vi "UHR-Fleezers Control (host) - 12.7e.vi"() -> ()   [LabVIEW 2012] (continued)
          tunnel: w4325 -> [w4338 w4370]
          tunnel: w4324 -> [w4337 w4369]
          tunnel: [w4336 w4368] -> w4322
          tunnel: [w4335 w4367] -> w4321
          tunnel: [w4333 w4354] -> w4319
          tunnel: [w4332 w4353] -> w4318
          tunnel: w4317 -> [w4333 w4359]
          tunnel: w4316 -> [w4332 w4362]
          tunnel: w4313 -> [_ _]
          frame False {
            w4334 = TRUE ("AI to FIFO")
            n2469 = xnode "Read/Write Control"("FPGA VI Reference In"=w4338, "error in"=w4337, "AI to FIFO"=w4334, "APD to FIFO"=w4334, "Start scan (MCL)"=w4334) -> ("FPGA VI Reference Out"=w4336:T20, "error out"=w4335:errorcluster)
          }
          frame True {
            w4366 = TRUE ("AI to FIFO")
            n2470 = local read "Scan steps (MCL)"() -> (w4345:u64)
            n2471 = local read "Scan lines (y)"() -> (w4341:u64)
            n2472 = local read "Fast Scan Dir"() -> (w4352:bool)
            n2473 = local read "Actual MCL Inc (V)"() -> (w4342:dbl)
            n2474 = Decrement(x=w4341) -> (x-1=w4340:u64)
            n2475 = Decrement(x=w4345) -> (x-1=w4344:u64)
            n2476 = Multiply(x=w4342, y=w4340) -> (x*y=w4339:dbl)
            n2477 = Divide(x=w4339, y=2.0) -> (x/y=w4349:dbl)
            n2478 = Multiply(x=w4342, y=w4344) -> (x*y=w4343:dbl)
            n2479 = Divide(x=w4343, y=2.0) -> (x/y=w4348:dbl)
            n2480 = Select(t=w4348, s=w4352, f=w4349) -> (s? t:f=w4347:dbl)
            n2481 = Select(t=w4349, s=w4352, f=w4348) -> (s? t:f=w4351:dbl)
            n2482 = Subtract(x=w4359, y=w4351) -> (x-y=w4350:dbl)
            n2483 = Subtract(x=w4362, y=w4347) -> (x-y=w4346:dbl)
            n2484 = local read "2D or 1D Scan"() -> (w4364:bool)
            n2485 = Not(x=w4352) -> (.not. x?=w4358:bool)
            n2486 = Not(x=w4364) -> (.not. x?=w4360:bool)
            n2487 = And(x=w4352, y=w4360) -> (x .and. y?=w4361:bool)
            n2488 = And(x=w4360, y=w4358) -> (x .and. y?=w4363:bool)
            n2489 = Select(t=w4362, s=w4363, f=w4346) -> (s? t:f=w4353:dbl)
            n2490 = Select(t=w4359, s=w4361, f=w4350) -> (s? t:f=w4354:dbl)
            n2491 = call "Volt to I16.vi"("Voltage In"=w4354) -> ("I16 Voltage Out"=w4357:i16)
            n2492 = call "Volt to I16.vi"("Voltage In"=w4353) -> ("I16 Voltage Out"=w4356:i16)
            n2493 = xnode "Read/Write Control"("FPGA VI Reference In"=w4370, "error in"=w4369, "AI to FIFO"=w4366, "APD to FIFO"=w4366, "Start scan (MCL)"=w4366, "AO1"=w4357, "AO2"=w4356) -> ("FPGA VI Reference Out"=w4368:T20, "error out"=w4367:errorcluster)
          }
        }
        "Initial Y" <- w4319
        "Initial X" <- w4318
        n2494 = local write "Tab Control 6"(T3."Imaging" ("Tab Control 6")) -> ()
        "wait to reset values" <- w4320
      }
    }
    n2495 = local read "APD Elements/DMA read"() -> (w3477:u32)
    n2496 = local read "Trap AI Elements/DMA read"() -> (w3694:u32)
    n2497 = xnode "Get APD Data"("FPGA VI Reference In"=w3633, "error in"=w3632, "Number of Elements"=w3477, "Timeout (ms)"=-1) -> ("Data"=w3663:u32[], "Elements Remaining"=→"APD FIFO Elements Remaining":u32)  [unwired: 2 out]
    n2498 = local read "Trap Pos Elements/DMA read"() -> (w3629:u32)
    n2499 = xnode "Invoke Method"("FPGA VI Reference In"=w3633, "error in"=w3632, "Number of Elements"=w3629, "Timeout (ms)"=-1) -> ("Data"=w3593:u16[], "Elements Remaining"=→"Trap Pos FIFO El Remaining":u32)  [unwired: 2 out]
    n2500 = xnode "Get Trap Data"("FPGA VI Reference In"=w3633, "error in"=w3632, "Number of Elements"=w3694, "Timeout (ms)"=-1 ("Timeout")) -> ("FPGA VI Reference Out"=w3528:T20, "error out"=w3527:errorcluster, "Data"=w3594:i16[], "Elements Remaining"=w3816:u32)
    "FIFO El. Rem." <- w3816
    n2501 = local read "DMA Update Period (s)"() -> (w3695:dbl)
    n2502 = local read "Trap AI FIFO Depth"() -> (w3818:u32)
    n2503 = local read "Number of APDs"() -> (w3496:u8)
    n2504 = Decimate 1D Array(w3593) -> (w3590:u16[], w3592:u16[], w3591:u16[])
    n2505 = feedback #6(0.0) -> (w3622:dbl)
    n2506 = Add(x=w3695, y=w3622) -> (x+y=w3792:dbl)
    n2507 = feedback-in #6(w3792) -> ()
    n2508 = To Time Stamp(1:w3622) -> (0:w3621:timestamp)
    n2509 = Subtract(x=w3818, y=w3694) -> (x-y=w3817:u32)
    n2510 = To Unsigned Long Integer(number=w3590) -> (unsigned 32bit integer=w3589:u32[])
    n2511 = Join Numbers(hi=w3592, lo=w3591) -> ((hi.lo)=w3588:u32[])
    n2512 = Divide(x=w3816, y=w3817) -> (x/y=w3815:dbl)
    "Buffer Status" <- w3815
    n2513 = case "Deinterlace APD signals" shown="3, Default" w3496 {
      tunnel: [w3828 w3834] -> w3476
      tunnel: w3663 -> [w3829 w3833]
      tunnel: [w3827 w3832] -> w3475
      tunnel: [w3826 w3830] -> w3462
      frame 3, Default {
        n2514 = Decimate 1D Array "APD signals"(w3829) -> (w3828:u32[], w3827:u32[], w3826:u32[])
      }
      frame 2 {
        n2515 = Decimate 1D Array "APD signals"(w3833) -> (w3834:u32[], w3832:u32[])
        n2516 = Multiply(x=w3832, y=u32 0) -> (x*y=w3830:u32[])
      }
    }
    n2517 = Join Numbers(hi=w3589, lo=w3588) -> ((hi.lo)=w3582:u64[])
    n2518 = call "IR AOM word to freq - vec.vi"("Frequency Word In (double vec)"=w3582) -> ("Frequency Out"=w3628:dbl[])
    n2519 = Equal?(x=w3815, y=1.0) -> (x = y?=w3813:bool)
    n2520 = case "Alert buffer overflow" shown="True" w3813 {
      frame False {
      }
      frame True {
        n2521 = call <vilib>:"Beep.vi"() -> ()  [unwired: 3 in, 9 out]
        "Overflow (data lost)" <- TRUE ("Overflow (data lost)")
      }
    }
    n2522 = Decimate 1D Array(w3628) -> (w3627:dbl[], w3626:dbl[])
    n2523 = Build Array(w3627, w3626) -> (w3625:dbl[][])
    n2524 = Bundle(w3476, w3475, w3462) -> (w3480:cluster{u32[], u32[], u32[]})  [unwired: 1 in]
    n2525 = Build Array(w3476, w3475, w3462) -> (w3753:u32[][])
    n2526 = for {
      tunnel: w3476 -> [w3824] mode=indexing
      n2527 = call "Smart Buffer (DBL) 1.vi"("new element [write]"=w3824, "mode"=T21."write") -> ()  [unwired: 4 in, 6 out]
    }
    n2528 = local read "APD Integration Time (s)"() -> (w3491:dbl)
    n2529 = To Double Precision Float(number=w3753) -> (double precision float=w3754:dbl[][])
    n2530 = feedback #7 "APD3"(w3462) -> (w3463:u32[])
    n2531 = feedback #8 "APD2"(w3475) -> (w3651:u32[])
    n2532 = feedback #9 "APD1"(w3476) -> (w3752:u32[])
    n2533 = Build Array (concatenate)(w3651, w3475) -> (w3650:u32[])
    n2534 = Build Array (concatenate)(w3463, w3462) -> (w3464:u32[])
    n2535 = Build Array (concatenate)(w3752, w3476) -> (w3749:u32[])
    n2536 = for {
      tunnel: w3475 -> [w3823] mode=indexing
      n2537 = call "Smart Buffer (DBL) 2.vi"("new element [write]"=w3823, "mode"=T21."write") -> ()  [unwired: 4 in, 6 out]
    }
    n2538 = Array Size(array=w3749) -> (size(s)=w3746:i32)
    n2539 = Array Size(array=w3476) -> (size(s)=w3748:i32)
    n2540 = Multiply(x=w3748, y="APD Ave N") -> (x*y=w3747:dbl)
    n2541 = Greater?(x=w3746, y=w3747) -> (0:w3750:bool)
    n2542 = Bundle("APD 1", "APD 2", "APD 3") -> (w3786:cluster{string, string, string})  [unwired: 1 out]
    n2543 = local read "Trap Sets"() -> (w3693:u32)
    n2544 = case shown="True" w3750 {
      tunnel: w3749 -> [w4126 w4135]
      tunnel: [w4126 w4133] -> w3700
      tunnel: w3747 -> [_ w4128]
      tunnel: w3746 -> [_ w4134]
      tunnel: w3650 -> [w4125 w4132]
      tunnel: [w4125 w4131] -> w3648
      tunnel: w3464 -> [w4124 w4130]
      tunnel: [w4124 w4127] -> w3492
      frame False {
      }
      frame True {
        n2545 = Subtract(x=w4134, y=w4128) -> (x-y=w4129:dbl)
        n2546 = Array Subset "APD3"(array=w4130, index=w4129, length=w4128) -> (w4127:u32[])
        n2547 = Array Subset "APD2"(array=w4132, index=w4129, length=w4128) -> (w4131:u32[])
        n2548 = Array Subset "APD1"(array=w4135, index=w4129, length=w4128) -> (w4133:u32[])
      }
    }
    n2549 = feedback-in #7(w3492) -> ()
    n2550 = feedback-in #8(w3648) -> ()
    n2551 = feedback-in #9(w3700) -> ()
    n2552 = Cluster To Array(cluster=w3786) -> (array=w3783:string[])
    n2553 = for "APD" {
      tunnel: w3754 -> [w4382] mode=indexing
      tunnel: w3491 -> [w4389]
      tunnel: [w4385] -> w3652 mode=indexing
      tunnel: "APD Disp. Scale" -> [w4386]
      tunnel: w3783 -> [w4384] mode=indexing
      tunnel: "APD Disp. Downsample" -> [w4380]
      tunnel: [w4383] -> w3782
      workers-P: _ -> [_]
      tunnel: w3621 -> [w4379]
      n2554 = call "integrate 1D array interval - double.vi"("Ave N"=w4380, "Array In"=w4382) -> ("Array Out"=w4381:dbl[])  [unwired: 1 out]
      n2555 = Multiply(x=w4389, y=w4380) -> (x*y=w4383:dbl)
      n2556 = Divide(x=w4381, y=w4386) -> (x/y=w4387:dbl[])
      n2557 = Bundle By Name("t0"=w4379, "Y"=w4387, "dt"=w4383) -> (w4388:waveform(dbl))  [unwired: 1 out]
      n2558 = Set Waveform Attribute(5:w4384, 6:"NI_ChannelName" ("name"), 7:w4388) -> (3:w4385:waveform(dbl))  [unwired: 1 in, 2 out]
    }
    "APD Display Period (s)" <- w3782
    n2559 = Reciprocal(x=w3782) -> (1/x=→"APD Display Freq. (Hz)":dbl)
    n2560 = case "Deinterlace trap data, average down PSD" shown="2" w3693 {
      tunnel: w3594 -> [w4407 w4472]
      tunnel: [w4404 w4469] -> w3686
      tunnel: [w4407 w4471] -> w3585
      tunnel: "Detector Type" -> [w4406 w4467]
      tunnel: [w4405 w4470] -> w3685
      tunnel: [w4403 w4468] -> w3790
      frame 1, Default {
        n2561 = Divide(x=w4407, y=3276.7) -> (x/y=w4408:dbl[])
        n2562 = Decimate 1D Array(w4408) -> (w4417:dbl[], w4416:dbl[], w4415:dbl[], w4414:dbl[], w4413:dbl[], w4412:dbl[], w4411:dbl[], w4410:dbl[])
        n2563 = case shown="\"IR-QPD + PSD + FB-QPD position\"" w4406 {
          tunnel: w4417 -> [w4441 w4466]
          tunnel: w4416 -> [w4440 w4465]
          tunnel: w4415 -> [w4425 w4443]
          tunnel: w4414 -> [w4426 w4453]
          tunnel: w4413 -> [w4439 w4464]
          tunnel: w4412 -> [w4438 w4463]
          tunnel: w4411 -> [w4422 w4444]
          tunnel: w4410 -> [w4421 w4442]
          tunnel: [w4420 w4450] -> w4405
          tunnel: [w4419 w4449] -> w4404
          tunnel: [w4418 w4448] -> w4403
          frame "IR-QPD + PSD + FB-QPD", Default {
            w4418 = 0  # Channel pattern
            n2564 = Divide(x=w4441, y=w4426) -> (x/y=w4428:dbl[])
            n2565 = Divide(x=w4440, y=w4426) -> (x/y=w4427:dbl[])
            n2566 = Divide(x=w4439, y=w4422) -> (x/y=w4424:dbl[])
            n2567 = Divide(x=w4438, y=w4421) -> (x/y=w4423:dbl[])
            n2568 = Build Array(w4428, w4427, w4426, w4425, w4424, w4423, w4422, w4421) -> (w4419:dbl[][])
            n2569 = Bundle("T1 Y", "T1 X", "T1 Sum", "FB Sum", "PSD Y", "PSD X", "PSD Y Sum", "PSD X Sum") -> (w4437:T44)  [unwired: 1 out]
            n2570 = Cluster To Array(cluster=w4437) -> (array=w4420:string[])
          }
          frame "IR-QPD + PSD + FB-QPD position" {
            w4448 = 3  # Channel pattern
            n2571 = Negate(x=w4444) -> (-x=w4445:dbl[])
            n2572 = Divide(x=w4466, y=w4453) -> (x/y=w4455:dbl[])
            n2573 = Divide(x=w4465, y=w4453) -> (x/y=w4454:dbl[])
            n2574 = Divide(x=w4464, y=w4444) -> (x/y=w4452:dbl[])
            n2575 = Divide(x=w4463, y=w4445) -> (x/y=w4451:dbl[])
            n2576 = Build Array(w4455, w4454, w4453, w4442, w4443, w4452, w4451, w4444) -> (w4449:dbl[][])
            n2577 = Bundle("T1 Y", "T1 X", "T1 Sum", "FB X", "FB Sum", "PSD Y", "PSD X", "PSD Y Sum") -> (w4462:T44)  [unwired: 1 out]
            n2578 = Cluster To Array(cluster=w4462) -> (array=w4450:string[])
          }
        }
      }
      frame 2 {
        n2579 = case shown="\"IR-QPD + PSD + FB-QPD X position\", Default" w4467 {
          tunnel: w4472 -> [w4534 w4606 w4677]
          tunnel: [w4473 w4597 w4608] -> w4471
          tunnel: [w4500 w4588 w4655] -> w4470
          tunnel: [w4499 w4551 w4622] -> w4469
          tunnel: [w4493 w4586 w4653] -> w4468
          frame "IR-QPD + PSD + FB-QPD" {
            w4493 = 1  # Channel pattern
            # "time average x2 the 4th signal and the 4 psd signals (detection laser)"
            # "deinterlace 3 signals from qpd"
            n2580 = Decimate 1D Array(w4534) -> (w4533:i16[], w4532:i16[], w4498:i16[], w4531:i16[], w4521:i16[], w4519:i16[], w4518:i16[], w4516:i16[])
            n2581 = Decimate 1D Array(w4498) -> (w4497:i16[], w4496:i16[])
            n2582 = Decimate 1D Array(w4533) -> (w4530:i16[], w4502:i16[])
            n2583 = Decimate 1D Array(w4532) -> (w4529:i16[], w4527:i16[])
            n2584 = Decimate 1D Array(w4531) -> (w4528:i16[], w4526:i16[])
            n2585 = call "downsample 1D array - double.vi"("Ave N"=2.0, "Array In"=w4521) -> ("Array Out"=w4520:dbl[])  [unwired: 1 out]
            n2586 = call "downsample 1D array - double.vi"("Ave N"=2.0, "Array In"=w4519) -> ("Array Out"=w4501:dbl[])  [unwired: 1 out]
            n2587 = call "downsample 1D array - double.vi"("Ave N"=2.0, "Array In"=w4518) -> ("Array Out"=w4517:dbl[])  [unwired: 1 out]
            n2588 = call "downsample 1D array - double.vi"("Ave N"=2.0, "Array In"=w4516) -> ("Array Out"=w4515:dbl[])  [unwired: 1 out]
            n2589 = Interleave 1D Arrays(w4530, w4529, w4528, w4502, w4527, w4526, w4497, w4496, w4520, w4501, w4517, w4515) -> (w4514:dbl[])
            n2590 = Divide(x=w4514, y=3276.7) -> (x/y=w4513:dbl[])
            n2591 = Decimate 1D Array(w4513) -> (w4512:dbl[], w4511:dbl[], w4510:dbl[], w4509:dbl[], w4508:dbl[], w4507:dbl[], w4495:dbl[], w4494:dbl[], w4506:dbl[], w4505:dbl[], w4504:dbl[], w4503:dbl[])
            n2592 = Divide(x=w4512, y=w4510) -> (x/y=w4480:dbl[])
            n2593 = Divide(x=w4511, y=w4510) -> (x/y=w4479:dbl[])
            n2594 = Divide(x=w4509, y=w4507) -> (x/y=w4478:dbl[])
            n2595 = Divide(x=w4508, y=w4507) -> (x/y=w4477:dbl[])
            n2596 = Divide(x=w4506, y=w4504) -> (x/y=w4476:dbl[])
            n2597 = Divide(x=w4505, y=w4503) -> (x/y=w4475:dbl[])
            n2598 = Build Array(w4480, w4479, w4510, w4478, w4477, w4507, w4495, w4494, w4476, w4475, w4504, w4503) -> (w4499:dbl[][])
            n2599 = Bundle("T1 Y", "T1 X", "T1 Sum", "T2 Y", "T2 X", "T2 Sum", "T1 FB Sum", "T2 FB Sum", "PSD Y", "PSD X", "PSD Y Sum", "PSD X Sum") -> (w4481:T45)  [unwired: 1 out]
            n2600 = To Word Integer(number=w4514) -> (16bit integer=w4473:i16[])
            n2601 = Cluster To Array(cluster=w4481) -> (array=w4500:string[])
          }
          frame "IR-QPD + PSD + FB-QPD X position", Default {
            w4586 = 2  # Channel pattern
            # "time average x2 the 3 psd signals (detection laser)"
            # "deinterlace 3 signals from qpds"
            n2602 = Decimate 1D Array(w4606) -> (w4605:i16[], w4604:i16[], w4587:i16[], w4603:i16[], w4549:i16[], w4546:i16[], w4543:i16[], w4574:i16[])
            n2603 = Select(t=i16 -1, s="Flip X Sign", f=i16 1) -> (s? t:f=w4539:i16)
            n2604 = Multiply(x=w4604, y=w4539) -> (x*y=w4540:i16[])
            n2605 = Decimate 1D Array(w4587) -> (w4572:i16[], w4570:i16[])
            n2606 = Decimate 1D Array(w4605) -> (w4602:i16[], w4589:i16[])
            n2607 = Decimate 1D Array(w4540) -> (w4601:i16[], w4599:i16[])
            n2608 = Decimate 1D Array(w4603) -> (w4600:i16[], w4598:i16[])
            n2609 = Decimate 1D Array(w4574) -> (w4573:i16[], w4571:i16[])
            n2610 = call "downsample 1D array - I16.vi"("Ave N"=2.0, "Array In"=w4549) -> ("Array Out"=w4547:i16[])  [unwired: 1 in]
            n2611 = call "downsample 1D array - I16.vi"("Ave N"=2.0, "Array In"=w4543) -> ("Array Out"=w4541:i16[])  [unwired: 1 in]
            n2612 = call "downsample 1D array - I16.vi"("Ave N"=2.0, "Array In"=w4546) -> ("Array Out"=w4544:i16[])  [unwired: 1 in]
            n2613 = Interleave 1D Arrays(w4602, w4601, w4600, w4589, w4599, w4598, w4573, w4572, w4571, w4570, w4547, w4544, w4541) -> (w4597:i16[])
            n2614 = Divide(x=w4597, y=3276.7) -> (x/y=w4596:dbl[])
            n2615 = Decimate 1D Array(w4596) -> (w4595:dbl[], w4594:dbl[], w4593:dbl[], w4592:dbl[], w4591:dbl[], w4590:dbl[], w4562:dbl[], w4560:dbl[], w4559:dbl[], w4557:dbl[], w4556:dbl[], w4555:dbl[], w4552:dbl[])
            n2616 = Negate(x=w4552) -> (-x=w4550:dbl[])
            n2617 = Divide(x=w4556, y=w4552) -> (x/y=w4554:dbl[])
            n2618 = Divide(x=w4555, y=w4550) -> (x/y=w4553:dbl[])
            n2619 = Divide(x=w4595, y=w4593) -> (x/y=w4578:dbl[])
            n2620 = Divide(x=w4594, y=w4593) -> (x/y=w4577:dbl[])
            n2621 = Divide(x=w4592, y=w4590) -> (x/y=w4576:dbl[])
            n2622 = Divide(x=w4591, y=w4590) -> (x/y=w4575:dbl[])
            n2623 = Divide(x=w4562, y=w4560) -> (x/y=w4561:dbl[])
            n2624 = Divide(x=w4559, y=w4557) -> (x/y=w4558:dbl[])
            n2625 = Build Array(w4578, w4577, w4593, w4576, w4575, w4590, w4561, w4560, w4558, w4557, w4554, w4553, w4552) -> (w4551:dbl[][])
            n2626 = Bundle("T1 Y", "T1 X", "T1 Sum", "T2 Y", "T2 X", "T2 Sum", "T1 FB X", "T1 FB Sum", "T2 FB X", "T2 FB Sum", "PSD Y", "PSD X", "PSD Y Sum") -> (w4579:T46)  [unwired: 1 out]
            n2627 = Cluster To Array(cluster=w4579) -> (array=w4588:string[])
          }
          frame "IR-QPD + PSD + FB-QPD XY positions" {
            w4653 = 4  # Channel pattern
            # "time average x2 the 3 psd signals (detection laser)"
            # "deinterlace 3 signals from qpds"
            n2628 = Decimate 1D Array(w4677) -> (w4676:i16[], w4675:i16[], w4654:i16[], w4674:i16[], w4620:i16[], w4666:i16[], w4665:i16[], w4642:i16[])
            n2629 = Decimate 1D Array "Feedback Sum"(w4654) -> (w4638:i16[], w4636:i16[])
            n2630 = Decimate 1D Array "QPD Y"(w4676) -> (w4673:i16[], w4656:i16[])
            n2631 = Decimate 1D Array "QPD X"(w4675) -> (w4672:i16[], w4670:i16[])
            n2632 = Decimate 1D Array "Feedback Y"(w4620) -> (w4619:i16[], w4618:i16[])
            n2633 = Decimate 1D Array "QPD Sum"(w4674) -> (w4671:i16[], w4669:i16[])
            n2634 = Decimate 1D Array "Feedback X"(w4642) -> (w4639:i16[], w4637:i16[])
            n2635 = call "downsample 1D array - double.vi"("Ave N"=2.0, "Array In"=w4666) -> ("Array Out"=w4641:dbl[])  [unwired: 1 out]
            n2636 = call "downsample 1D array - double.vi"("Ave N"=2.0, "Array In"=w4665) -> ("Array Out"=w4640:dbl[])  [unwired: 1 out]
            n2637 = Interleave 1D Arrays(w4673, w4672, w4671, w4656, w4670, w4669, w4619, w4639, w4638, w4618, w4637, w4636, w4641, w4640) -> (w4664:dbl[])
            n2638 = Divide(x=w4664, y=3276.7) -> (x/y=w4663:dbl[])
            n2639 = Decimate 1D Array(w4663) -> (w4662:dbl[], w4661:dbl[], w4660:dbl[], w4659:dbl[], w4658:dbl[], w4657:dbl[], w4615:dbl[], w4629:dbl[], w4613:dbl[], w4614:dbl[], w4627:dbl[], w4611:dbl[], w4625:dbl[], w4623:dbl[])
            n2640 = Negate(x=w4623) -> (-x=w4621:dbl[])
            n2641 = Divide(x=w4625, y=w4621) -> (x/y=w4624:dbl[])
            n2642 = Divide(x=w4614, y=w4611) -> (x/y=w4610:dbl[])
            n2643 = Divide(x=w4615, y=w4613) -> (x/y=w4612:dbl[])
            n2644 = Divide(x=w4662, y=w4660) -> (x/y=w4646:dbl[])
            n2645 = Divide(x=w4661, y=w4660) -> (x/y=w4645:dbl[])
            n2646 = Divide(x=w4659, y=w4657) -> (x/y=w4644:dbl[])
            n2647 = Divide(x=w4658, y=w4657) -> (x/y=w4643:dbl[])
            n2648 = Divide(x=w4629, y=w4613) -> (x/y=w4628:dbl[])
            n2649 = Divide(x=w4627, y=w4611) -> (x/y=w4626:dbl[])
            n2650 = Build Array(w4646, w4645, w4660, w4644, w4643, w4657, w4612, w4628, w4613, w4610, w4626, w4611, w4624, w4623) -> (w4622:dbl[][])
            n2651 = Bundle("T1 Y", "T1 X", "T1 Sum", "T2 Y", "T2 X", "T2 Sum", "T1 FB Y", "T1 FB X", "T1 FB Sum", "T2 FB Y", "T2 FB X", "T2 FB Sum", "PSD X", "PSD Y Sum") -> (w4609:T47)  [unwired: 1 out]
            n2652 = To Word Integer(number=w4664) -> (16bit integer=w4608:i16[])
            n2653 = Cluster To Array(cluster=w4609) -> (array=w4655:string[])
          }
        }
      }
    }
    "AI labels" <- w3685
    n2654 = local read "APD Integration Time (s)"() -> (w3658:dbl)
    n2655 = Array Size(array=w3700) -> (size(s)=w3745:i32)
    n2656 = call <vilib>:"Std Deviation and Variance.vi"("X"=w3648) -> ("standard deviation"=w3647:dbl)  [unwired: 1 in, 2 out]
    n2657 = Add Array Elements(numeric array=w3648) -> (sum=w3649:u32)
    n2658 = Add Array Elements(numeric array=w3700) -> (sum=w3755:u32)
    n2659 = call <vilib>:"Std Deviation and Variance.vi"("X"=w3700) -> ("standard deviation"=w3699:dbl)  [unwired: 1 in, 2 out]
    n2660 = Divide(x=w3647, y=w3491) -> (x/y=w3644:dbl)
    "Rate sigma (Hz) 2" <- w3644
    n2661 = Multiply(x=w3491, y=w3745) -> (x*y=w3493:dbl)
    "Int. Time (s)" <- w3493
    n2662 = Divide(x=w3649, y=w3493) -> (x/y=w3645:dbl)
    "APD 2 Rate (Hz)" <- w3645
    n2663 = Multiply(x="APD Disp. Scale", y=w3652) -> (x*y=w3660:waveform(dbl)[])
    n2664 = Divide(x=w3755, y=w3493) -> (x/y=w3697:dbl)
    "APD 1 Rate (Hz)" <- w3697
    n2665 = Divide(x=w3699, y=w3491) -> (x/y=w3698:dbl)
    "Rate sigma (Hz)" <- w3698
    n2666 = Divide(x=w3644, y=w3645) -> (x/y=→"Sigma/Mean 2":dbl)
    n2667 = Multiply(x="APD Disp. Downsample", y=w3658) -> (x*y=w3656:dbl)
    n2668 = Divide(x=w3698, y=w3697) -> (x/y=→"Sigma/Mean":dbl)
    n2669 = Divide(x=w3660, y=w3656) -> (x/y=w3483:waveform(dbl)[])
    n2670 = Index Array(array=w3483, index=0) -> (element=w3641:waveform(dbl))
    n2671 = Index Array(array=w3483, index=1) -> (element=w3639:waveform(dbl))
    n2672 = Index Array(array=w3483, index=2) -> (element=w3485:waveform(dbl))
    n2673 = Subtract(x=w3641, y="APD 1 Offset") -> (x-y=w3637:waveform(dbl))
    n2674 = Subtract(x=w3639, y="APD 2 Offset") -> (x-y=w3636:waveform(dbl))
    n2675 = Subtract(x=w3485, y="APD 3 Offset") -> (x-y=w3482:waveform(dbl))
    n2676 = Add Array Elements(numeric array=w3492) -> (sum=w3495:u32)
    n2677 = call <vilib>:"Std Deviation and Variance.vi"("X"=w3492) -> ("standard deviation"=w3494:dbl)  [unwired: 1 in, 2 out]
    n2678 = Build Array(w3637, w3636, w3482) -> (→"APD Chart":waveform(dbl)[])
    n2679 = Divide(x=w3495, y=w3493) -> (x/y=w3489:dbl)
    "APD 3 Rate (Hz)" <- w3489
    n2680 = Divide(x=w3494, y=w3491) -> (x/y=w3490:dbl)
    "Rate sigma (Hz) 3" <- w3490
    n2681 = Divide(x=w3490, y=w3489) -> (x/y=→"Sigma/Mean 3":dbl)
    n2682 = local read "Data Period (s)"() -> (w3544:dbl)
    n2683 = local read "BD 1 Frequency 2 (MHz)"() -> (w3577:dbl)
    n2684 = local read "BD 1 Frequency 1 (MHz)"() -> (w3578:dbl)
    n2685 = Decimate 1D Array(w3585) -> (w3609:i16[], w3608:i16[], w3606:i16[], w3605:i16[])  [unwired: 9 out]
    n2686 = Multiply(x=w3544, y="Trap Pos. Disp. Downsample") -> (x*y=w3542:dbl)
    n2687 = Divide(x=w3609, y=w3608) -> (x/y=w3610:dbl[])
    n2688 = Divide(x=w3606, y=w3605) -> (x/y=w3607:dbl[])
    n2689 = local read "AOM X Cal (nm/MHz)"() -> (w3575:dbl)
    n2690 = Split 1D Array(array=w3610, index="N El. to Ave.") -> (second subarray=w3613:dbl[])  [unwired: 1 out]
    n2691 = Split 1D Array(array=w3607, index="N El. to Ave.") -> (second subarray=w3612:dbl[])  [unwired: 1 out]
    n2692 = Multiply(x=w3544, y="Trap Disp. Downsample") -> (x*y=w3623:dbl)
    "Display Period (s)" <- w3623
    n2693 = for "Trap AI" {
      tunnel: [w4402] -> w3469 mode=indexing
      tunnel: w3621 -> [w4393]
      tunnel: "Trap Disp. Downsample" -> [w4400]
      tunnel: w3686 -> [w4398] mode=indexing
      tunnel: w3544 -> [w4397]
      tunnel: w3685 -> [w4396] mode=indexing
      tunnel: [w4395] -> w3655 mode=indexing
      tunnel: w3623 -> [w4394]
      workers-P: _ -> [_]
      n2694 = Bundle By Name("Y"=w4398, "dt"=w4397) -> (w4399:waveform(dbl))  [unwired: 1 out]
      n2695 = Set Waveform Attribute(5:w4396, 6:"NI_ChannelName" ("name"), 7:w4399) -> (3:w4395:waveform(dbl))  [unwired: 1 in, 2 out]
      n2696 = call "downsample 1D array - double.vi"("Ave N"=w4400, "Array In"=w4398) -> ("Array Out"=w4401:dbl[])  [unwired: 1 out]
      n2697 = Bundle By Name(cluster=w4395, "t0"=w4393, "Y"=w4401, "dt"=w4394) -> (w4402:waveform(dbl))
    }
    n2698 = Bundle("BD 1 Frequency 1 (MHz)"=w3578, "BD 1 Frequency 2 (MHz)"=w3577) -> (w3579:T48)  [unwired: 1 out]
    n2699 = call-poly <vilib>:"Mean.vi"("X"=w3612) -> ("mean"=w3600:dbl)  [unwired: 1 out]
    n2700 = call-poly <vilib>:"Mean.vi"("X"=w3613) -> ("mean"=w3601:dbl)  [unwired: 1 out]
    n2701 = Reciprocal(x=w3623) -> (1/x=→"Trap Disp. Freq. (Hz)":dbl)
    n2702 = Cluster To Array(cluster=w3579) -> (array=w3576:dbl[])
    n2703 = local read "Trap X AI1 (DMA)"() -> (w3611:T13)
    n2704 = local read "Data points/scans (MCL)"() -> (w3765:dbl)
    n2705 = To Fixed-Point(number=w3600) -> (fixed-point=w3598:fxp<+/-,16,1>)  [unwired: 1 in]
    n2706 = To Fixed-Point(number=w3601) -> (fixed-point=w3599:fxp<+/-,16,1>)  [unwired: 1 in]
    n2707 = Bundle("Trap 1 Pos.", "Trap 2 Pos.") -> (w3620:cluster{string, string})  [unwired: 1 out]
    n2708 = Bundle By Name(cluster=w3611, "Set 1"=w3599, "Set 2"=w3598) -> (→"Trap X AI1 (DMA)":T13)
    n2709 = Cluster To Array(cluster=w3620) -> (array=w3617:string[])
    n2710 = Unbundle(w3480) -> (w3481:u32[])  [unwired: 2 out]
    n2711 = Select(t=-1.0, s="Negate Y Axis", f=1.0) -> (s? t:f=w3561:dbl)
    n2712 = for "Trap Position" {
      tunnel: w3625 -> [w3994] mode=indexing
      tunnel: "Trap Pos. Disp. Downsample" -> [w3993]
      tunnel: w3542 -> [w3991]
      tunnel: w3621 -> [w3990]
      tunnel: w3617 -> [w3988] mode=indexing
      tunnel: [w3987] -> w3531 mode=indexing
      tunnel: w3576 -> [w3985] mode=indexing
      tunnel: w3575 -> [w3983]
      tunnel: w3561 -> [w3982]
      n2713 = call "downsample 1D array - double.vi"("Ave N"=w3993, "Array In"=w3994) -> ("Array Out"=w3992:dbl[])  [unwired: 1 out]
      n2714 = Subtract(x=w3992, y=w3985) -> (x-y=w3986:dbl[])
      n2715 = Multiply(x=w3983, y=w3986) -> (x*y=w3984:dbl[])
      n2716 = Multiply(x=w3982, y=w3984) -> (x*y=w3981:dbl[])
      n2717 = Bundle By Name("Y"=w3981, "dt"=w3991, "t0"=w3990) -> (w3989:waveform(dbl))  [unwired: 1 out]
      n2718 = Set Waveform Attribute(5:w3988, 6:"NI_ChannelName" ("name"), 7:w3989) -> (3:w3987:waveform(dbl))  [unwired: 1 in, 2 out]
    }
    n2719 = To Double Precision Float(number=w3481) -> (double precision float=w3683:dbl[])
    n2720 = local read "Display Period (s)"() -> (w3672:dbl)
    n2721 = Increment(x=w3765) -> (x+1=w3766:dbl)
    n2722 = Index Array(array=w3531, index=0) -> (element=w3535:waveform(dbl))
    n2723 = Index Array(array=w3531, index=1) -> (element=w3530:waveform(dbl))
    n2724 = feedback #10(w3766) -> (w3769:dbl)
    n2725 = Select(t=0, s=w3756, f=w3769) -> (s? t:f=w3762:dbl)
    n2726 = Array Size(array=w3683) -> (size(s)=w3768:i32)
    n2727 = Build Array (concatenate)(w3652, w3469) -> (w3474:waveform(dbl)[])
    "All Signals" <- w3474
    n2728 = Add(x=w3768, y=w3762) -> (x+y=w3763:dbl)
    n2729 = Unbundle By Name(w3535) -> ("Y"=w3536:dbl[])
    n2730 = Divide(x="Bead Sep. Int. Time (s)", y=w3672) -> (x/y=w3571:dbl)
    n2731 = Add(x=w3536, y="FB Trap Pos Offset") -> (x+y=w3534:dbl[])
    "T1 x pos data" <- w3534
    n2732 = Greater?(x=w3763, y=w3765) -> (0:w3764:bool)
    n2733 = feedback #11(w3534) -> (w3573:dbl[])
    n2734 = Build Array (concatenate)(w3534, w3573) -> (w3572:dbl[])
    n2735 = Bundle By Name(cluster=w3535, "Y"=w3534) -> (w3533:waveform(dbl))
    n2736 = Select(t=w3762, s=w3764, f=w3763) -> (s? t:f=w3761:dbl)
    n2737 = feedback-in #10(w3761) -> ()
    n2738 = local read "MCL Scanning"() -> (w3759:bool)
    n2739 = Bundle(w3533, w3530) -> (w3529:cluster{waveform(dbl), waveform(dbl)})  [unwired: 1 out]
    n2740 = Index Array(array=w3469, index="index 1") -> (element=w3468:waveform(dbl))
    n2741 = Index Array(array=w3469, index="index 2") -> (element=w3473:waveform(dbl))
    n2742 = Split 1D Array(array=w3572, index=w3571) -> (first subarray=w3565:dbl[])  [unwired: 1 out]
    n2743 = feedback-in #11(w3565) -> ()
    n2744 = Unbundle By Name(w3468) -> ("Y"=w3467:dbl[])
    n2745 = Unbundle By Name(w3473) -> ("Y"=w3472:dbl[])
    n2746 = Not(x=w3764) -> (.not. x?=w3758:bool)
    n2747 = Cluster To Array(cluster=w3529) -> (array=w3505:waveform(dbl)[])
    "Trap Positions" <- w3505
    n2748 = call-poly <vilib>:"Mean.vi"("X"=w3565) -> ("mean"=w3564:dbl)  [unwired: 1 out]
    "Mean T1 Position (nm)" <- w3564
    n2749 = Subtract(x=w3565, y=w3564) -> (x-y=w3570:dbl[])
    n2750 = Square(x=w3570) -> (x^2=w3569:dbl[])
    n2751 = And(x=w3758, y=w3759) -> (x .and. y?=w3760:bool)
    n2752 = call-poly <vilib>:"Mean.vi"("X"=w3569) -> ("mean"=w3568:dbl)  [unwired: 1 out]
    n2753 = call-poly <vilib>:"Mean.vi"("X"=w3467) -> ("mean"=→"Trap 1 sum mean":dbl)  [unwired: 1 out]
    n2754 = call-poly <vilib>:"Mean.vi"("X"=w3472) -> ("mean"=→"Trap 2 sum mean":dbl)  [unwired: 1 out]
    n2755 = Square Root(x=w3568) -> (sqrt(x)=w3567:dbl)
    n2756 = Or(x=w3760, y=w3756) -> (x .or. y?=w3757:bool)
    n2757 = Equal?(x="Tab Control 6", y=T38."High Res Display") -> (x = y?=w3689:bool)
    n2758 = Multiply(x=10.0, y=w3567) -> (x*y=→"Trap 1 Position RMS (A)":dbl)
    n2759 = case "For displaying the high resolution display (no downsampling)" shown="True" w3689 {
      tunnel: w3655 -> [_ w4014]
      frame False {
      }
      frame True {
        n2760 = Index Array(array=w4014, index="High Res. Display") -> (element=w4015:waveform(dbl))
        n2761 = call <vilib>:"Std Deviation and Variance.vi"("X"=w4015) -> ("mean"=w4022:dbl, "standard deviation"=w4027:dbl)  [unwired: 1 in, 1 out]
        "Mean Intensity" <- w4022
        "Sigma" <- w4027
        n2762 = Subtract(x=w4015, y=w4022) -> (x-y=w4021:waveform(dbl))
        n2763 = Select(t=w4021, s="Subtract mean", f=w4015) -> (s? t:f=→"1 Channel":waveform(dbl))
        n2764 = Divide(x=w4027, y=w4022) -> (x/y=→"Sigma/Mean":dbl)
        n2765 = feedback #12(1) -> (w4016:i32)
        n2766 = Greater Or Equal?(x=w4016, y="Slow mean N ave.") -> (x >= y?=w4029:bool)
        n2767 = Increment(x=w4016) -> (x+1=w4031:i32)
        n2768 = Select(t=1, s=w4029, f=w4031) -> (s? t:f=w4018:i32)
        n2769 = feedback-in #12(w4018) -> ()
        n2770 = feedback #13() -> (w4019:waveform(dbl))  [unwired: 1 out]
        n2771 = case shown="Default" w4016 {
          tunnel: [w4034 w4037] -> w4020
          tunnel: w4019 -> [w4036 _]
          tunnel: w4015 -> [w4035 w4037]
          frame Default {
            n2772 = call-poly <vilib>:"Append Waveforms.vi"("waveform B"=w4035, "waveform A"=w4036) -> ("waveform out"=w4034:waveform(dbl))  [unwired: 1 in, 8 out]
          }
          frame 1 {
          }
        }
        n2773 = feedback-in #13(w4020) -> ()
        n2774 = case shown="True" w4029 {
          tunnel: w4020 -> [_ w4033]
          frame False {
          }
          frame True {
            n2775 = call-poly <vilib>:"Mean.vi"("X"=w4033) -> ("mean"=→"Slow mean":dbl)  [unwired: 1 out]
          }
        }
      }
    }
    n2776 = case "For plotting results of scanning MCL (fluorescence and detection laser images)" shown="True" w3757 {
      tunnel: w3756 -> [_ w4143]
      tunnel: w3765 -> [_ _]
      tunnel: w3655 -> [_ w4270]
      tunnel: w3634 -> [_ w4178]
      tunnel: w3480 -> [_ w4149]
      frame False {
      }
      frame True {
        w4159 = u32 0 items=["Horizontal", "Vertical", "Central", "1st Diagonal", "2nd Diagonal"] ("Type of Symmetry")
        w4185 = u32 0 items=["Horizontal", "Vertical", "Central", "1st Diagonal", "2nd Diagonal"] ("Type of Symmetry")
        w4209 = u32 0 items=["Horizontal", "Vertical", "Central", "1st Diagonal", "2nd Diagonal"] ("Type of Symmetry")
        w4212 = u32 0 items=["Horizontal", "Vertical", "Central", "1st Diagonal", "2nd Diagonal"] ("Type of Symmetry")
        w4241 = u32 0 items=["Horizontal", "Vertical", "Central", "1st Diagonal", "2nd Diagonal"] ("Type of Symmetry")
        n2777 = Unbundle(w4149) -> (w4148:u32[], w4146:u32[], w4144:u32[])
        n2778 = To Double Precision Float(number=w4148) -> (double precision float=w4147:dbl[])
        n2779 = To Double Precision Float(number=w4146) -> (double precision float=w4145:dbl[])
        n2780 = To Double Precision Float(number=w4144) -> (double precision float=w4136:dbl[])
        n2781 = Index Array(array=w4270, index=10) -> (element=w4276:waveform(dbl))
        n2782 = Index Array(array=w4270, index=11) -> (element=w4273:waveform(dbl))
        n2783 = local read "Cycles/step (MCL)"() -> (w4226:u64)
        n2784 = Index Array(array=w4270, index="Channel") -> (element=w4272:waveform(dbl))
        n2785 = Unbundle(w4178) -> ("New Image"=w4177:T2, "New Image"=w4176:T2, "New Image"=w4150:T2, "New Image"=w4151:T2, "New Image"=w4152:T2)
        n2786 = local read "Scan steps (MCL)"() -> (w4139:u64)
        n2787 = Unbundle By Name(w4276) -> ("Y"=w4228:dbl[])
        n2788 = Unbundle By Name(w4273) -> ("Y"=w4230:dbl[])
        n2789 = local read "Scan lines (y)"() -> (w4140:u64)
        n2790 = local read "N APD Samp/step"() -> (w4142:dbl)
        n2791 = Unbundle By Name(w4272) -> ("Y"=w4235:dbl[])
        n2792 = call "downsample 1D array - double.vi"("Ave N"=w4226, "Array In"=w4228) -> ("Array Out"=w4227:dbl[])  [unwired: 1 out]
        n2793 = call "downsample 1D array - double.vi"("Ave N"=w4226, "Array In"=w4230) -> ("Array Out"=w4229:dbl[])  [unwired: 1 out]
        n2794 = call "downsample 1D array - double.vi"("Ave N"=w4226, "Array In"=w4235) -> ("Array Out"=w4234:dbl[])  [unwired: 1 out]
        n2795 = Multiply(x=w4139, y=u64 2) -> (x*y=w4141:u64)
        n2796 = feedback #14(w4145) -> (w4203:dbl[])
        n2797 = Build Array (concatenate)(w4203, w4145) -> (w4202:dbl[])
        n2798 = feedback #15(w4136) -> (w4137:dbl[])
        n2799 = Build Array (concatenate)(w4137, w4136) -> (w4138:dbl[])
        n2800 = Select(t=w4145, s=w4143, f=w4202) -> (s? t:f=w4187:dbl[])
        n2801 = feedback-in #14(w4187) -> ()
        n2802 = Select(t=w4136, s=w4143, f=w4138) -> (s? t:f=w4161:dbl[])
        n2803 = feedback-in #15(w4161) -> ()
        n2804 = feedback #16(w4147) -> (w4296:dbl[])
        n2805 = Build Array (concatenate)(w4296, w4147) -> (w4278:dbl[])
        n2806 = Select(t=w4147, s=w4143, f=w4278) -> (s? t:f=w4282:dbl[])
        n2807 = feedback-in #16(w4282) -> ()
        n2808 = feedback #17(w4227) -> (w4284:dbl[])
        n2809 = Build Array (concatenate)(w4284, w4227) -> (w4275:dbl[])
        n2810 = feedback #18(w4234) -> (w4294:dbl[])
        n2811 = Build Array (concatenate)(w4294, w4234) -> (w4293:dbl[])
        n2812 = feedback #19(w4229) -> (w4286:dbl[])
        n2813 = Build Array (concatenate)(w4286, w4229) -> (w4287:dbl[])
        n2814 = Select(t=w4227, s=w4143, f=w4275) -> (s? t:f=w4231:dbl[])
        n2815 = feedback-in #17(w4231) -> ()
        n2816 = Select(t=w4234, s=w4143, f=w4293) -> (s? t:f=w4233:dbl[])
        n2817 = feedback-in #18(w4233) -> ()
        n2818 = Select(t=w4229, s=w4143, f=w4287) -> (s? t:f=w4232:dbl[])
        n2819 = feedback-in #19(w4232) -> ()
        n2820 = call "integrate 1D array interval - double.vi"("Ave N"=w4142, "Array In"=w4187) -> ("Array Out"=w4198:dbl[])  [unwired: 1 out]
        n2821 = call "integrate 1D array interval - double.vi"("Ave N"=w4142, "Array In"=w4161) -> ("Array Out"=w4172:dbl[])  [unwired: 1 out]
        n2822 = call "integrate 1D array interval - double.vi"("Ave N"=w4142, "Array In"=w4282) -> ("Array Out"=w4281:dbl[])  [unwired: 1 out]
        n2823 = Array Size(array=w4198) -> (size(s)=w4199:i32)
        n2824 = Array Size(array=w4172) -> (size(s)=w4173:i32)
        n2825 = Array Size(array=w4281) -> (size(s)=w4283:i32)
        n2826 = Multiply(x=w4140, y=w4141) -> (x*y=w4201:u64)
        n2827 = Multiply(x=w4140, y=w4141) -> (x*y=w4175:u64)
        n2828 = Multiply(x=w4140, y=w4141) -> (x*y=w4291:u64)
        n2829 = Subtract(x=w4201, y=w4199) -> (x-y=w4192:u64)
        n2830 = call-poly <vilib>:"Mean.vi"("X"=w4198) -> ("mean"=w4189:dbl)  [unwired: 1 out]
        n2831 = Subtract(x=w4175, y=w4173) -> (x-y=w4166:u64)
        n2832 = call-poly <vilib>:"Mean.vi"("X"=w4172) -> ("mean"=w4163:dbl)  [unwired: 1 out]
        n2833 = Subtract(x=w4291, y=w4283) -> (x-y=w4225:u64)
        n2834 = call-poly <vilib>:"Mean.vi"("X"=w4281) -> ("mean"=w4222:dbl)  [unwired: 1 out]
        n2835 = call-poly <vilib>:"Mean.vi"("X"=w4231) -> ("mean"=w4215:dbl)  [unwired: 1 out]
        n2836 = call-poly <vilib>:"Mean.vi"("X"=w4233) -> ("mean"=w4220:dbl)  [unwired: 1 out]
        n2837 = call-poly <vilib>:"Mean.vi"("X"=w4232) -> ("mean"=w4218:dbl)  [unwired: 1 out]
        n2838 = Initialize Array(1.0 ("element"), w4192) -> (w4188:dbl[])
        n2839 = Initialize Array(1.0 ("element"), w4166) -> (w4162:dbl[])
        n2840 = Initialize Array(1.0 ("element"), w4225) -> (w4216:dbl[])
        n2841 = Multiply(x=w4188, y=w4189) -> (x*y=w4190:dbl[])
        n2842 = Multiply(x=w4162, y=w4163) -> (x*y=w4164:dbl[])
        n2843 = Multiply(x=w4216, y=w4222) -> (x*y=w4223:dbl[])
        n2844 = Multiply(x=w4216, y=w4218) -> (x*y=w4219:dbl[])
        n2845 = Multiply(x=w4216, y=w4220) -> (x*y=w4221:dbl[])
        n2846 = Multiply(x=w4216, y=w4215) -> (x*y=w4217:dbl[])
        n2847 = Build Array (concatenate)(w4198, w4190) -> (w4200:dbl[])
        n2848 = Build Array (concatenate)(w4172, w4164) -> (w4174:dbl[])
        n2849 = Build Array (concatenate)(w4281, w4223) -> (w4290:dbl[])
        n2850 = Build Array (concatenate)(w4231, w4217) -> (w4285:dbl[])
        n2851 = Build Array (concatenate)(w4233, w4221) -> (w4289:dbl[])
        n2852 = Build Array (concatenate)(w4232, w4219) -> (w4288:dbl[])
        n2853 = Reshape Array(w4200, w4140, w4141) -> (w4196:dbl[][])
        n2854 = Reshape Array(w4174, w4140, w4141) -> (w4170:dbl[][])
        n2855 = Reshape Array(w4290, w4140, w4141) -> (w4268:dbl[][])
        n2856 = Reshape Array(w4285, w4140, w4141) -> (w4251:dbl[][])
        n2857 = Reshape Array(w4289, w4140, w4141) -> (w4243:dbl[][])
        n2858 = Reshape Array(w4288, w4140, w4141) -> (w4258:dbl[][])
        n2859 = Array Subset(array=w4196, index (col)=0 ("index"), length (col)=w4139) -> (w4195:dbl[][])  [unwired: 2 in]
        n2860 = Array Subset(array=w4196, index (col)=w4139) -> (w4193:dbl[][])  [unwired: 3 in]
        n2861 = Array Subset(array=w4170, index (col)=0 ("index"), length (col)=w4139) -> (w4169:dbl[][])  [unwired: 2 in]
        n2862 = Array Subset(array=w4170, index (col)=w4139) -> (w4167:dbl[][])  [unwired: 3 in]
        n2863 = Array Subset(array=w4258, index (col)=0 ("index"), length (col)=w4139) -> (w4263:dbl[][])  [unwired: 2 in]
        n2864 = Array Subset(array=w4258, index (col)=w4139) -> (w4261:dbl[][])  [unwired: 3 in]
        n2865 = Array Subset(array=w4268, index (col)=0 ("index"), length (col)=w4139) -> (w4267:dbl[][])  [unwired: 2 in]
        n2866 = Array Subset(array=w4268, index (col)=w4139) -> (w4265:dbl[][])  [unwired: 3 in]
        n2867 = Array Subset(array=w4243, index (col)=0 ("index"), length (col)=w4139) -> (w4249:dbl[][])  [unwired: 2 in]
        n2868 = Array Subset(array=w4243, index (col)=w4139) -> (w4247:dbl[][])  [unwired: 3 in]
        n2869 = Array Subset(array=w4251, index (col)=0 ("index"), length (col)=w4139) -> (w4256:dbl[][])  [unwired: 2 in]
        n2870 = Array Subset(array=w4251, index (col)=w4139) -> (w4254:dbl[][])  [unwired: 3 in]
        n2871 = for {
          tunnel: w4195 -> [w4300] mode=indexing
          tunnel: [w4299] -> w4194 mode=indexing
          workers-P: _ -> [_]
          n2872 = Reverse 1D Array(array=w4300) -> (reversed array=w4299:dbl[])
        }
        n2873 = for {
          tunnel: w4169 -> [w4298] mode=indexing
          tunnel: [w4297] -> w4168 mode=indexing
          workers-P: _ -> [_]
          n2874 = Reverse 1D Array(array=w4298) -> (reversed array=w4297:dbl[])
        }
        n2875 = for {
          tunnel: w4263 -> [w4306] mode=indexing
          tunnel: [w4305] -> w4262 mode=indexing
          workers-P: _ -> [_]
          n2876 = Reverse 1D Array(array=w4306) -> (reversed array=w4305:dbl[])
        }
        n2877 = for {
          tunnel: w4267 -> [w4308] mode=indexing
          tunnel: [w4307] -> w4266 mode=indexing
          workers-P: _ -> [_]
          n2878 = Reverse 1D Array(array=w4308) -> (reversed array=w4307:dbl[])
        }
        n2879 = for {
          tunnel: w4249 -> [w4302] mode=indexing
          tunnel: [w4301] -> w4248 mode=indexing
          workers-P: _ -> [_]
          n2880 = Reverse 1D Array(array=w4302) -> (reversed array=w4301:dbl[])
        }
        n2881 = for {
          tunnel: w4256 -> [w4304] mode=indexing
          tunnel: [w4303] -> w4255 mode=indexing
          workers-P: _ -> [_]
          n2882 = Reverse 1D Array(array=w4304) -> (reversed array=w4303:dbl[])
        }
        n2883 = Index Array(array=w4268, index (row)=0) -> (element=→"Waveform Graph":dbl[])  [unwired: 1 in]
        n2884 = Add(x=w4194, y=w4193) -> (x+y=w4180:dbl[][])
        n2885 = Add(x=w4168, y=w4167) -> (x+y=w4154:dbl[][])
        n2886 = Add(x=w4262, y=w4261) -> (x+y=w4260:dbl[][])
        n2887 = Add(x=w4266, y=w4265) -> (x+y=w4240:dbl[][])
        n2888 = Add(x=w4248, y=w4247) -> (x+y=w4246:dbl[][])
        n2889 = Add(x=w4255, y=w4254) -> (x+y=w4253:dbl[][])
        n2890 = Divide(x=w4246, y=2) -> (x/y=w4244:dbl[][])
        n2891 = Divide(x=w4260, y=2) -> (x/y=w4205:dbl[][])
        n2892 = To Single Precision Float(number=w4240) -> (single precision float=w4239:sgl[][])
        n2893 = To Single Precision Float(number=w4180) -> (single precision float=w4184:sgl[][])
        n2894 = To Single Precision Float(number=w4154) -> (single precision float=w4158:sgl[][])
        n2895 = Divide(x=w4253, y=2) -> (x/y=w4207:dbl[][])
        n2896 = Transpose 2D Array(2D array=w4244) -> (transposed array=→"Data map":dbl[][])
        n2897 = To Single Precision Float(number=w4205) -> (single precision float=w4211:sgl[][])
        n2898 = To Single Precision Float(number=w4207) -> (single precision float=w4208:sgl[][])
        n2899 = call "IMAQ ArrayToImage"("Image Pixels (Float)"=w4239, "Image"=w4177) -> ("Image Out"=w4242:T2)  [unwired: 8 in, 1 out]
        n2900 = call "IMAQ ArrayToImage"("Image Pixels (Float)"=w4184, "Image"=w4176) -> ("Image Out"=w4186:T2)  [unwired: 8 in, 1 out]
        n2901 = call "IMAQ ArrayToImage"("Image Pixels (Float)"=w4158, "Image"=w4150) -> ("Image Out"=w4160:T2)  [unwired: 8 in, 1 out]
        n2902 = call "IMAQ ArrayToImage"("Image Pixels (Float)"=w4211, "Image"=w4151) -> ("Image Out"=w4213:T2)  [unwired: 8 in, 1 out]
        n2903 = call "IMAQ Symmetry"("Type of Symmetry"=w4241, "Image Src"=w4242) -> ("Image Dst Out"=w4237:T2)  [unwired: 3 in, 1 out]
        n2904 = call "IMAQ ArrayToImage"("Image Pixels (Float)"=w4208, "Image"=w4152) -> ("Image Out"=w4210:T2)  [unwired: 8 in, 1 out]
        n2905 = call "IMAQ Symmetry"("Type of Symmetry"=w4185, "Image Src"=w4186) -> ("Image Dst Out"=w4182:T2)  [unwired: 3 in, 1 out]
        n2906 = call "IMAQ Symmetry"("Type of Symmetry"=w4159, "Image Src"=w4160) -> ("Image Dst Out"=w4156:T2)  [unwired: 3 in, 1 out]
        n2907 = call "IMAQ Symmetry"("Type of Symmetry"=w4212, "Image Src"=w4213) -> ("Image Dst Out"=→"Detection Laser X":T2)  [unwired: 3 in, 1 out]
        n2908 = call "IMAQ Symmetry"("Type of Symmetry"=w4209, "Image Src"=w4210) -> ("Image Dst Out"=→"Detection Laser Y":T2)  [unwired: 3 in, 1 out]
        n2909 = call "IMAQ Set Simple Calibration"("Calibration Axis Info"=T39 {"Origin Pixel"={"X"=0.0, "Y"=0.0}, "Angle Relative to Horizontal (deg)"=0.0, "Axis Reference"=0}, "Grid Descriptor"=T40 {"X Step"=0.3, "Y Step"=0.3, "Unit"=enum."Undefined"}, "Image"=w4237) -> ("Calibrated Image"=→"APD 1":T2)  [unwired: 7 in, 1 out]
        n2910 = call "IMAQ Set Simple Calibration"("Calibration Axis Info"=T39 {"Origin Pixel"={"X"=0.0, "Y"=0.0}, "Angle Relative to Horizontal (deg)"=0.0, "Axis Reference"=0}, "Grid Descriptor"=T40 {"X Step"=0.3, "Y Step"=0.3, "Unit"=enum."Undefined"}, "Image"=w4182) -> ("Calibrated Image"=→"APD 2":T2)  [unwired: 7 in, 1 out]
        n2911 = call "IMAQ Set Simple Calibration"("Calibration Axis Info"=T39 {"Origin Pixel"={"X"=0.0, "Y"=0.0}, "Angle Relative to Horizontal (deg)"=0.0, "Axis Reference"=0}, "Grid Descriptor"=T40 {"X Step"=0.3, "Y Step"=0.3, "Unit"=enum."Undefined"}, "Image"=w4156) -> ("Calibrated Image"=→"APD 3":T2)  [unwired: 7 in, 1 out]
      }
    }
    n2912 = case "For computing FFTs for display" shown="True" "Compute FFT" {
      tunnel: w3655 -> [_ w4780]
      frame False {
      }
      frame True {
        n2913 = Build Array("FFT 1 Choice 1", "FFT 1 Choice 2", "FFT 2 Choice 1", "FFT 2 Choice 2") -> (w4773:u16[])
        n2914 = Array Size(array=w4780) -> (size(s)=w4779:i32)
        n2915 = feedback-in #20(w4773) -> ()
        n2916 = feedback #20(u16[] [100, 100, 100, 100]) -> (w4774:u16[])
        n2917 = feedback-in #21("# Spectra to Ave.") -> ()
        n2918 = feedback #21("# Spectra to Ave.") -> (w4771:dbl)
        n2919 = Not Equal?(x="# Spectra to Ave.", y=w4771) -> (x != y?=w4770:bool)
        n2920 = Not Equal?(x=w4773, y=w4774) -> (x != y?=w4772:bool)
        n2921 = feedback #22(1.0) -> (w4757:dbl)
        n2922 = Compound Arithmetic op=OR("Reset FFT", w4772, w4770) -> (w4755:bool)
        n2923 = Select(t=1.0, s=w4755, f=w4757) -> (s? t:f=w4759:dbl)
        n2924 = Greater?(x=w4759, y="# Spectra to Ave.") -> (0:w4778:bool)
        n2925 = Increment(x=w4759) -> (x+1=w4758:dbl)
        n2926 = feedback-in #22(w4758) -> ()
        n2927 = local read "DMA Update Period (s)"() -> (w4753:dbl)
        n2928 = Multiply(x="# Spectra to Ave.", y=w4753) -> (x*y=→"Ave. Time (s)":dbl)
        n2929 = Build Array(cluster{"f0":dbl, "df":dbl, "magnitude":dbl[]} {"f0"=0.0, "df"=0.0, "magnitude"=[]} ("PSD")) -> (w4762:cluster{"f0":dbl, "df":dbl, "magnitude":dbl[]}[])
        n2930 = Build Array(w4762, w4762, w4762, w4762) -> (w4764:T49)
        n2931 = feedback #23(w4764) -> (w4769:T49)
        n2932 = for {
          N: 4 -> [_]
          tunnel: w4773 -> [w4802] mode=indexing
          tunnel: w4780 -> [w4803]
          tunnel: w4779 -> [w4805]
          tunnel: w4755 -> [w4798]
          tunnel: w4778 -> [w4797]
          tunnel: "# Spectra to Ave." -> [w4796]
          tunnel: [w4795] -> w4768 mode=indexing
          tunnel: w4769 -> [w4800] mode=indexing
          tunnel: [w4799] -> w4756 mode=indexing
          tunnel: w4759 -> [w4794]
          n2933 = Less?(x=w4802, y=w4805) -> (x < y?=w4804:bool)
          n2934 = Index Array(array=w4803, index=w4802) -> (element=w4801:waveform(dbl))
          n2935 = case shown="True" w4804 {
            tunnel: w4801 -> [_ w4822]
            tunnel: w4800 -> [w4807 w4820]
            tunnel: [w4807 w4808] -> w4799
            tunnel: w4798 -> [_ w4819]
            tunnel: w4797 -> [_ w4812]
            tunnel: w4796 -> [_ w4811]
            tunnel: [cluster{"f0":dbl, "df":dbl, "magnitude":dbl[]} {"f0"=0.0, "df"=0.0, "magnitude"=[]} ("PSD") w4813] -> w4795
            tunnel: w4794 -> [_ w4810]
            frame False {
            }
            frame True {
              n2936 = call <vilib>:"Std Deviation and Variance.vi"("X"=w4822) -> ("mean"=w4823:dbl)  [unwired: 1 in, 2 out]
              n2937 = Subtract(x=w4822, y=w4823) -> (x-y=w4821:waveform(dbl))
              n2938 = xnode "Spectral Measurements"("Signals"=w4821) -> ("PSD"=w4815:cluster{"f0":dbl, "df":dbl, "magnitude":dbl[]})  [unwired: 1 in, 1 out]
              n2939 = case shown="False" w4819 {
                tunnel: w4820 -> [w4832 _]
                tunnel: [w4828 w4837] -> w4808
                tunnel: w4815 -> [w4831 w4838]
                tunnel: w4812 -> [w4830 _]
                frame False {
                  n2940 = Build Array (concatenate)(w4832, w4831) -> (w4829:cluster{"f0":dbl, "df":dbl, "magnitude":dbl[]}[])
                  n2941 = case shown="True" w4830 {
                    tunnel: w4829 -> [w4833 w4836]
                    tunnel: [w4833 w4834] -> w4828
                    frame False {
                    }
                    frame True {
                      n2942 = Delete From Array(array=w4836, index=0) -> (array with subset deleted=w4834:cluster{"f0":dbl, "df":dbl, "magnitude":dbl[]}[])  [unwired: 1 in, 1 out]
                    }
                  }
                }
                frame True {
                  n2943 = Build Array(w4838) -> (w4837:cluster{"f0":dbl, "df":dbl, "magnitude":dbl[]}[])
                }
              }
              n2944 = for {
                tunnel: w4808 -> [w4827] mode=indexing
                tunnel: [w4826] -> w4818 mode=indexing
                workers-P: _ -> [_]
                n2945 = Unbundle By Name(w4827) -> ("magnitude"=w4826:dbl[])
              }
              n2946 = Transpose 2D Array(2D array=w4818) -> (transposed array=w4817:dbl[][])
              n2947 = for {
                tunnel: w4817 -> [w4825] mode=indexing
                tunnel: [w4824] -> w4816 mode=indexing
                workers-P: _ -> [_]
                n2948 = Add Array Elements(numeric array=w4825) -> (sum=w4824:dbl)
              }
              n2949 = Select(t=w4811, s=w4812, f=w4810) -> (s? t:f=w4809:dbl)
              n2950 = Divide(x=w4816, y=w4809) -> (x/y=w4814:dbl[])
              n2951 = Bundle By Name(cluster=w4815, "magnitude"=w4814) -> (w4813:cluster{"f0":dbl, "df":dbl, "magnitude":dbl[]})
            }
          }
        }
        n2952 = case shown="True" w4755 {
          tunnel: w4756 -> [w4787 w4793]
          tunnel: [w4787 w4788] -> w4754
          frame False {
          }
          frame True {
            n2953 = Array Subset(array=w4793, index (row)=0 ("index"), length (row)=4 ("length"), index (col)=0 ("index"), length (col)=1 ("length")) -> (w4788:T49)
          }
        }
        n2954 = feedback-in #23(w4754) -> ()
        n2955 = Split 1D Array(array=w4768, index=2) -> (first subarray=→"FFT 1":cluster{"f0":dbl, "df":dbl, "magnitude":dbl[]}[], second subarray=→"FFT 2":cluster{"f0":dbl, "df":dbl, "magnitude":dbl[]}[])
      }
    }
    n2956 = Index Array(array=w3474, index=4) -> (element=w3709:waveform(dbl))
    n2957 = Index Array(array=w3474, index=7) -> (element=w3706:waveform(dbl))
    n2958 = Divide(x="T1 offset_x (mV)", y=1000.0) -> (x/y=w3710:dbl)
    n2959 = feedback-in #24("Calibration") -> ()
    n2960 = feedback #24(u16 1 ("Calibration")) -> (w3728:u16)
    n2961 = Divide(x="T2 offset_x (mV)", y=1000.0) -> (x/y=w3708:dbl)
    n2962 = case shown="2" "Calibration" {
      tunnel: "T1 alpha_x (nm/V)" -> [_ w4101 w4122]
      tunnel: "T1 kappa_x (pN/nm)" -> [_ _ w4112]
      tunnel: "T2 alpha_x (nm/V)" -> [_ w4100 w4120]
      tunnel: "T2 kappa_x (pN/nm)" -> [_ _ w4113]
      tunnel: w3709 -> [w4083 w4098 w4118]
      tunnel: w3706 -> [w4082 w4096 w4116]
      tunnel: [w4083 w4095 w4115] -> w3737
      tunnel: [w4082 w4094 w4114] -> w3736
      tunnel: ["T1 X (V)" ("Label.Text") "T1 X (nm)" ("Label.Text") "T1 X (pN)" ("Label.Text")] -> w3725
      tunnel: ["T2 X (V)" ("Label.Text") "T2 X (nm)" ("Label.Text") "T2 X (pN)" ("Label.Text")] -> w3724
      tunnel: ["Position (V)" ("Label.Text") "Position (nm)" ("Label.Text") "Force (pN)" ("Label.Text")] -> w3726
      tunnel: w3708 -> [_ w4086 w4105]
      tunnel: w3710 -> [_ w4089 w4107]
      tunnel: ["Mean (V)" ("Label.Text") "Mean (nm)" ("Label.Text") "Mean (pN)" ("Label.Text")] -> w3721
      tunnel: ["Difference (V)" ("Label.Text") "Difference (nm)" ("Label.Text") "Difference (pN)" ("Label.Text")] -> w3661
      frame 0, Default {
      }
      frame 1 {
        n2963 = Unbundle By Name(w4098) -> ("Y"=w4102:dbl[])
        n2964 = Unbundle By Name(w4096) -> ("Y"=w4087:dbl[])
        n2965 = Subtract(x=w4102, y=w4089) -> (x-y=w4090:dbl[])
        n2966 = Subtract(x=w4087, y=w4086) -> (x-y=w4088:dbl[])
        n2967 = Multiply(x=w4088, y=w4100) -> (x*y=w4097:dbl[])
        n2968 = Multiply(x=w4101, y=w4090) -> (x*y=w4099:dbl[])
        n2969 = Bundle By Name(cluster=w4096, "Y"=w4097) -> (w4094:waveform(dbl))
        n2970 = Bundle By Name(cluster=w4098, "Y"=w4099) -> (w4095:waveform(dbl))
      }
      frame 2 {
        n2971 = Unbundle By Name(w4118) -> ("Y"=w4123:dbl[])
        n2972 = Unbundle By Name(w4116) -> ("Y"=w4121:dbl[])
        n2973 = Subtract(x=w4121, y=w4105) -> (x-y=w4106:dbl[])
        n2974 = Subtract(x=w4123, y=w4107) -> (x-y=w4108:dbl[])
        n2975 = Compound Arithmetic op=MULTIPLY(w4106, w4120, w4113) -> (w4117:dbl[])
        n2976 = Compound Arithmetic op=MULTIPLY(w4112, w4122, w4108) -> (w4119:dbl[])
        n2977 = Bundle By Name(cluster=w4116, "Y"=w4117) -> (w4114:waveform(dbl))
        n2978 = Bundle By Name(cluster=w4118, "Y"=w4119) -> (w4115:waveform(dbl))
      }
    }
    n2979 = case shown="True" "Read Lateness and Rel Phase" {
      tunnel: w3528 -> [w4038 w4071]
      tunnel: w3527 -> [w4039 w4070]
      tunnel: [w4038 w4043] -> w3703
      tunnel: [w4039 w4042] -> w3702
      frame False {
      }
      frame True {
        n2980 = xnode "Read/Write Control"("FPGA VI Reference In"=w4071, "error in"=w4070) -> ("FPGA VI Reference Out"=w4045:T20, "error out"=w4044:errorcluster, "GI Relative phase"=→"GI relative phase":i16, "Relative phase"=→"Relative phase (AI1)":i16, "AI Late Counter"=→"Late Counter (AI1)":u8, "GI Late Counter"=→"GI Late Counter":u8, "MCL Late Counter"=→"MCL Late Counter":u8, "MCL Relative Phase"=→"Relative Phase (MCL)":i16, "APD Acq Relative Phase"=→"APD Acq Relative Phase":i16, "APD 1 Gate Relative Phase"=→"APD 1 Gate Relative Phase":i16, "APD 2 Gate Relative Phase"=→"APD 2 Gate Relative Phase":i16, "APD Acq Late Counter"=→"APD Acq Late Counter":u8, "APD 1 Gate Late Counter"=→"APD 1 Gate Late Counter":u8, "APD 2 Gate Late Counter"=→"APD 2 Gate Late Counter":u8, "Green FB Relative Phase"=→"Relative phase (Green FB)":i16, "GI Relative phase 2"=→"GI relative phase 2":i16, "GI Late Counter 2"=→"GI Late Counter 2":u8, "Trap Pos FIFO Timeout"=→"Trap Pos FIFO Timeout":u16, "Trap AI FIFO Timeout"=→"Trap AI FIFO Timeout":u16, "RI Late Counter"=→"RI Late Counter":u8, "RI Relative phase"=→"RI relative phase":i16, "Green Late Counter"=→"Green AI Late Counter":u8, "BI Late Counter (AO)"=→"Late Counter (BI AO)":u8, "Blue Late Counter (D)"=→"Late Counter (BI DO)":u8, "BI Relative phase (AO)"=→"Relative phase (BI AO)":i16, "BI Relative phase (D)"=→"Relative phase (BI DO)":i16)